vi "De_Band_HXRG.vi"(7 "Transpose":bool, 11 "IMAGE 2":i32[][](graph)=array1024x1024[1048576 elements]) -> (3 "IMAGE":dbl[][](graph))   [LabVIEW 2017]
uses:
  <vilib>/Analysis/baseanly.llb/Mean (DBL).vi
  <vilib>/Analysis/NI_AALBase.lvlib
panel:
  out "Waveform Graph 3":dbl[][](graph)
  out "Step #":i32
  out "IMAGE 3":i32[][](graph)
  out "Top Ref pixs":dbl[](array[numeric])
  out "Bottom Ref pixs":dbl[](array[numeric])
  out "Q3 avg":dbl=-0.8184616088867186
  out "Q3 RMS":dbl=19.25740971624928
  out "Q4 avg":dbl=1.3942337036132815
  out "Q4 RMS":dbl=26.97344260258525
  out "Q1 RMS":dbl=21.389760464347606
  out "Q1 avg":dbl=2.3578338623046875
  out "Q2  RMS":dbl=28.329968380841386
  out "Q2 avg":dbl=0.05986480712890625
  out "mean before":dbl=0.1424398422241211
  out "RMS before":dbl=23.67379491089448
  out "mean a fter":dbl=0.7448520660400391
  out "RMS  after":dbl=24.28217603569673
  in  "Array side Q3":u16(ring)=2 items=["Left", "Bottom", "Right", "Top"]
  in  "Array side Q4":u16(ring)=2 items=["Left", "Bottom", "Right", "Top"]
  in  "Array side Q1":u16(ring) items=["Left", "Bottom", "Right", "Top"]
  in  "Array side Q2":u16(ring) items=["Left", "Bottom", "Right", "Top"]
  out "Orig Array":i32[][](array[numeric])
  in  "Num Ref Pix":i32=5
  out "Sub Array":i32[][](array[numeric])
  # "right"
  # "left"
  # "left"
  # "right"
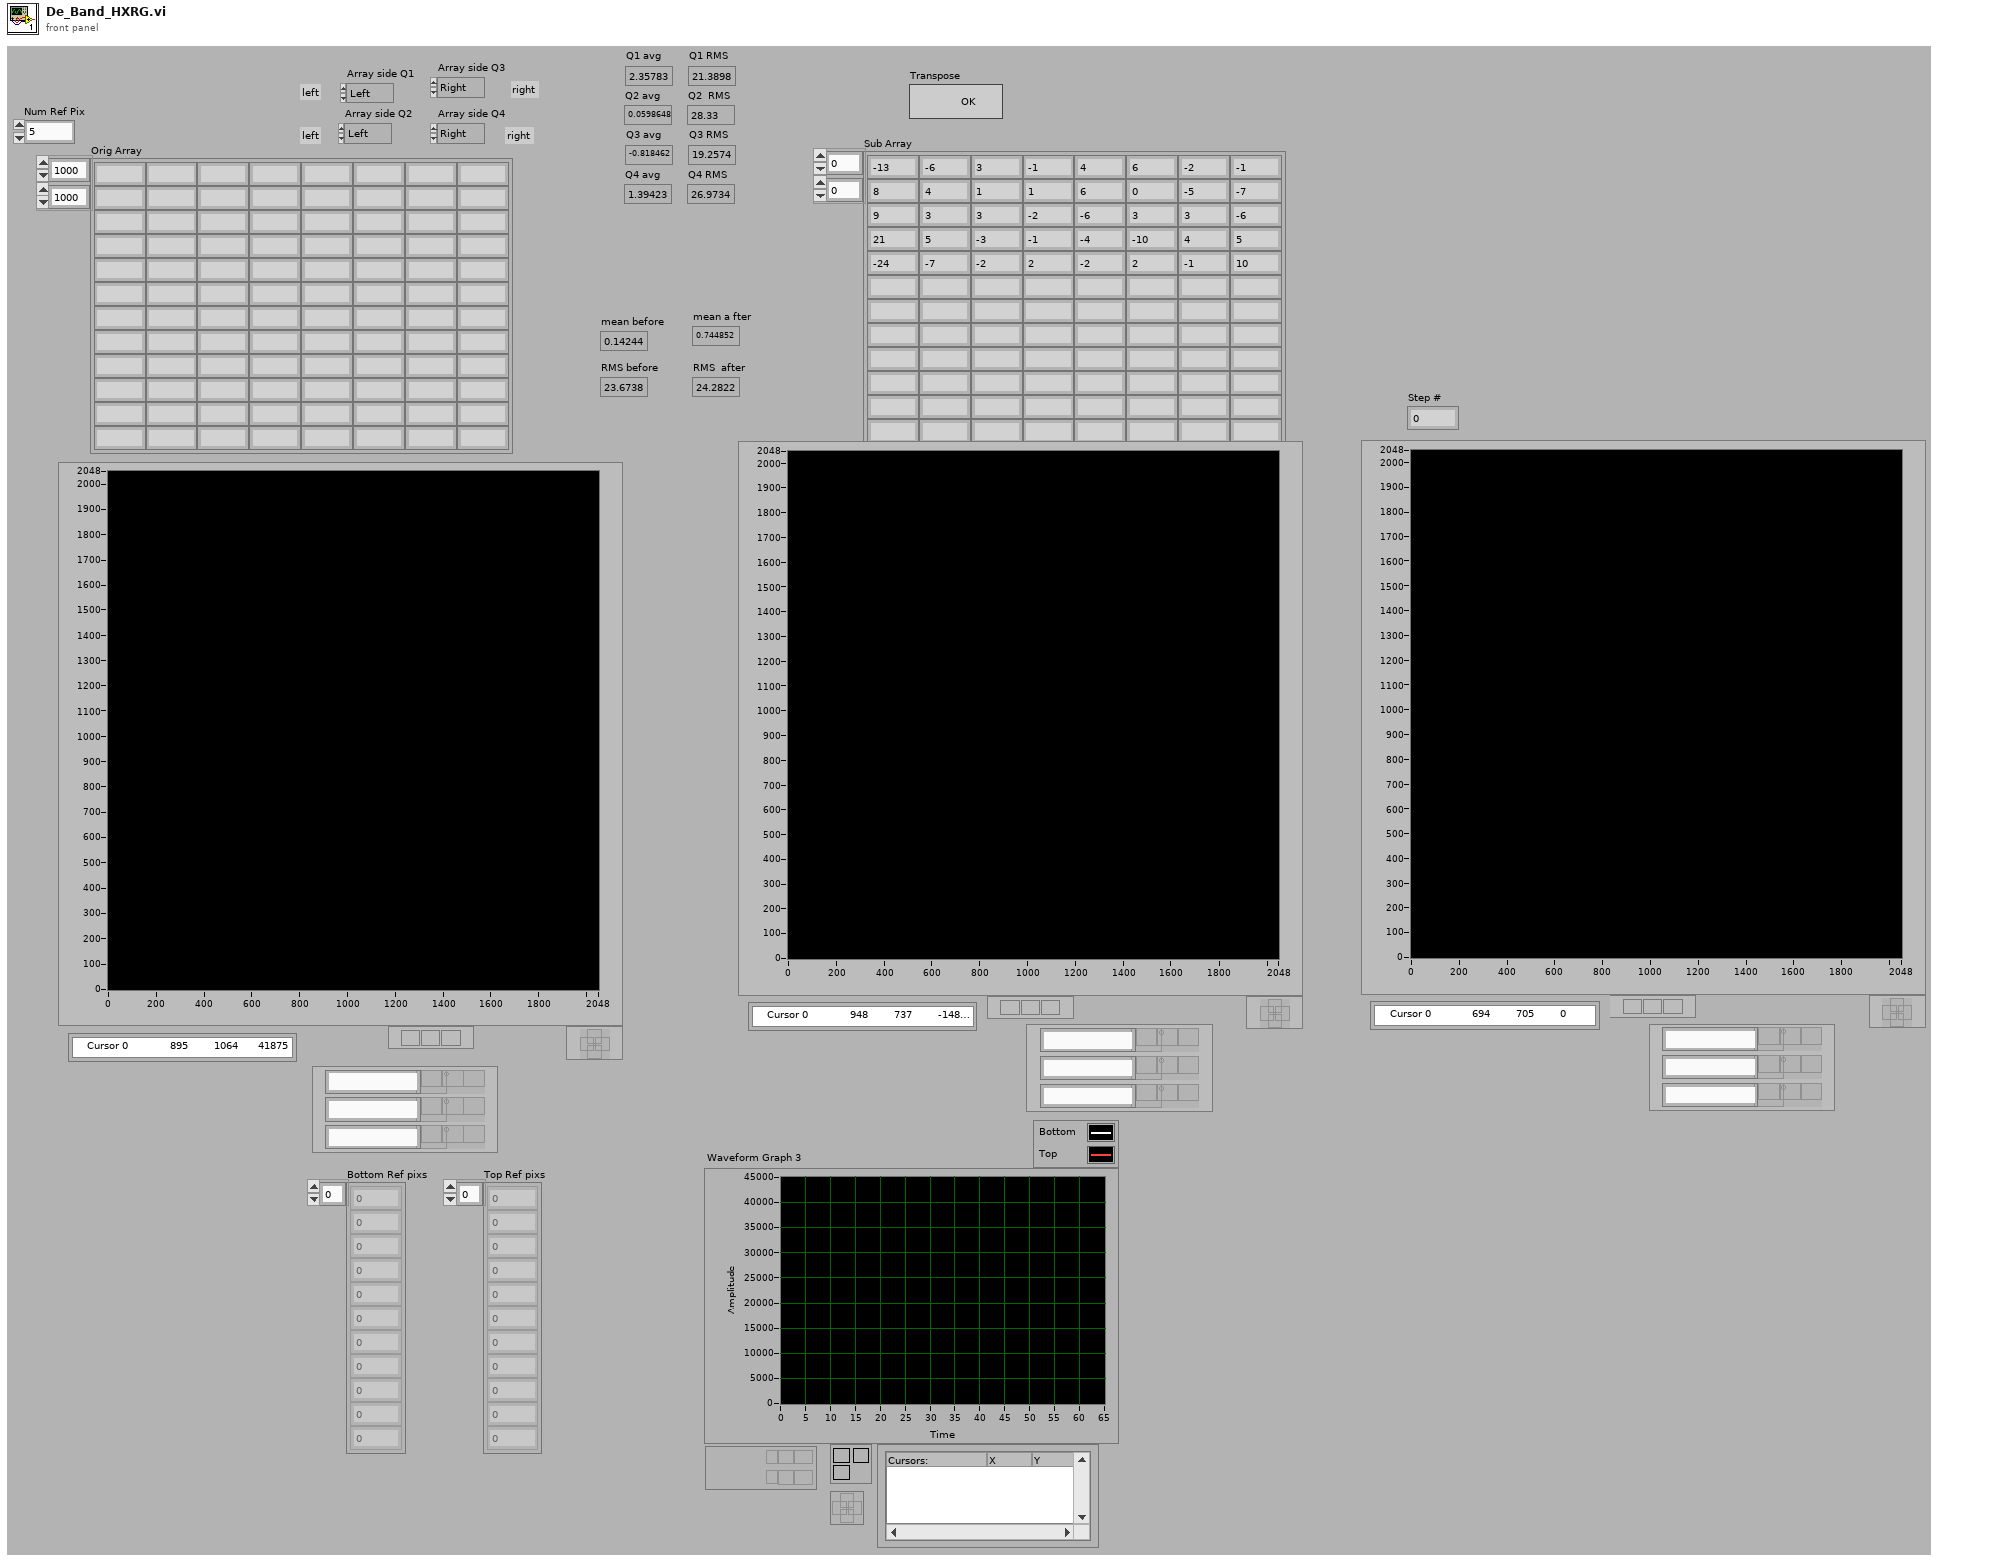
[diagram p1: front panel]
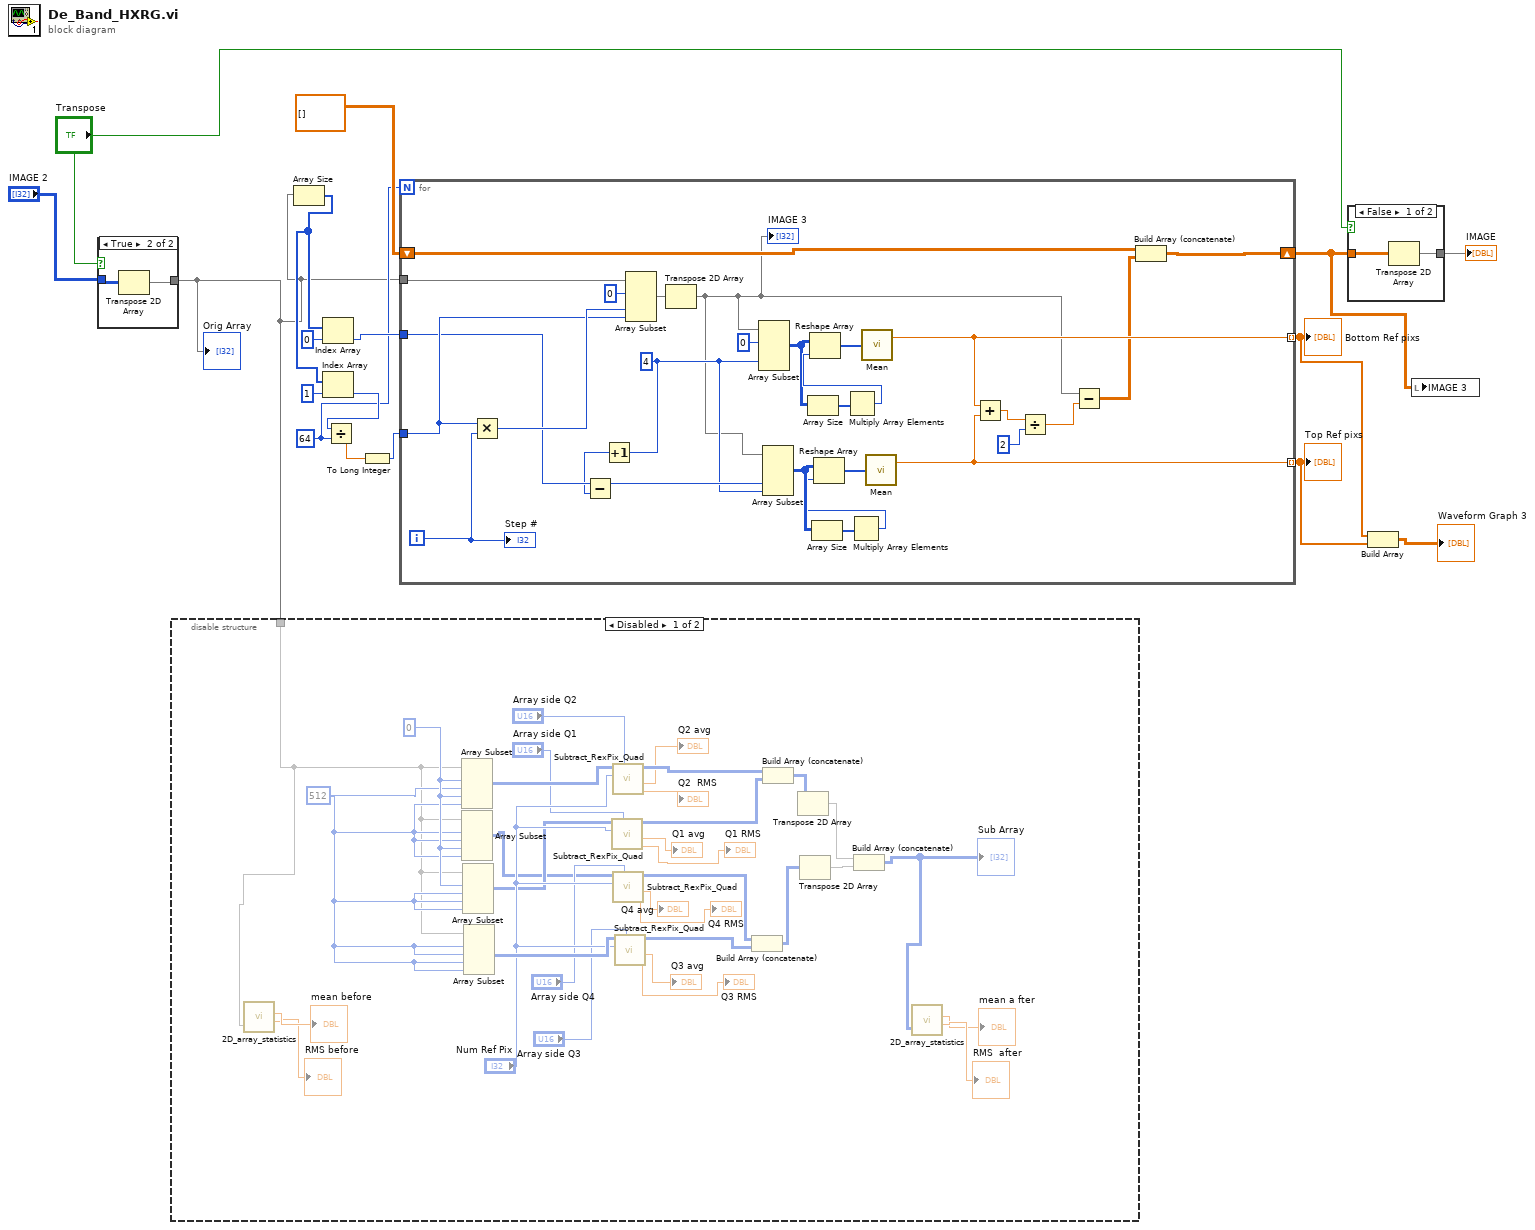
[diagram p0: block diagram]
diagram:
  w9 = 64 ("y")
  n1 = case shown="True" "Transpose" {
    tunnel: [w18 w19] -> w4
    tunnel: "IMAGE 2" -> [w18 w20]
    frame False {
    }
    frame True {
      n2 = Transpose 2D Array(2D array=w20) -> (transposed array=w19:i32[][])
    }
  }
  "Orig Array" <- w4
  n3 = disable-structure shown="Disabled" {
    disable-tunnel: w4 -> [w21 _]
    frame Disabled {
      w25 = 0
      w22 = 512
      n4 = call <userlib>:"2D_array_statistics.vi"("Array"=w21) -> ("mean 2"=→"mean before":dbl, "RMS 2"=→"RMS before":dbl)  [unwired: 2 in, 2 out]
      n5 = Array Subset(array=w21, index (row)=w25, length (row)=w22, index (col)=w25, length (col)=w22) -> (w49:i32[][])
      n6 = Array Subset(array=w21, index (row)=w22, length (row)=w22, index (col)=w25, length (col)=w22) -> (w23:i32[][])
      n7 = Array Subset(array=w21, index (row)=w25, length (row)=w22, index (col)=w22, length (col)=w22) -> (w24:i32[][])
      n8 = Array Subset(array=w21, index (row)=w22, length (row)=w22, index (col)=w22, length (col)=w22) -> (w47:i32[][])
      n9 = call <userlib>:"Subtract_RexPix_Quad.vi"("Array side"="Array side Q1", "Num Ref Pix"="Num Ref Pix", "Quad array"=w24) -> ("RMS 2"=→"Q1 RMS":dbl, "mean 2"=→"Q1 avg":dbl, "Quad array subtracted ref pixs"=w45:i32[][])  [unwired: 5 in, 1 out]
      n10 = call <userlib>:"Subtract_RexPix_Quad.vi"("Array side"="Array side Q2", "Num Ref Pix"="Num Ref Pix", "Quad array"=w49) -> ("RMS 2"=→"Q2  RMS":dbl, "mean 2"=→"Q2 avg":dbl, "Quad array subtracted ref pixs"=w48:i32[][])  [unwired: 5 in, 1 out]
      n11 = call <userlib>:"Subtract_RexPix_Quad.vi"("Array side"="Array side Q4", "Num Ref Pix"="Num Ref Pix", "Quad array"=w23) -> ("RMS 2"=→"Q4 RMS":dbl, "mean 2"=→"Q4 avg":dbl, "Quad array subtracted ref pixs"=w44:i32[][])  [unwired: 5 in, 1 out]
      n12 = call <userlib>:"Subtract_RexPix_Quad.vi"("Array side"="Array side Q3", "Num Ref Pix"="Num Ref Pix", "Quad array"=w47) -> ("RMS 2"=→"Q3 RMS":dbl, "mean 2"=→"Q3 avg":dbl, "Quad array subtracted ref pixs"=w43:i32[][])  [unwired: 5 in, 1 out]
      n13 = Build Array (concatenate)(w44, w43) -> (w50:i32[][])
      n14 = Build Array (concatenate)(w48, w45) -> (w51:i32[][])
      n15 = Transpose 2D Array(2D array=w51) -> (transposed array=w52:i32[][])
      n16 = Transpose 2D Array(2D array=w50) -> (transposed array=w53:i32[][])
      n17 = Build Array (concatenate)(w52, w53) -> (w34:i32[][])
      "Sub Array" <- w34
      n18 = call <userlib>:"2D_array_statistics.vi"("Array"=w34) -> ("mean 2"=→"mean a fter":dbl, "RMS 2"=→"RMS  after":dbl)  [unwired: 2 in, 2 out]
    }
    frame Enabled {
    }
  }
  n19 = Array Size(array=w4) -> (size(s)=w15:i32[])
  n20 = Index Array(array=w15, index=0) -> (element=w11:i32)
  n21 = Index Array(array=w15, index=1) -> (element=w14:i32)
  n22 = Divide(x=w14, y=w9) -> (x/y=w13:dbl)
  n23 = To Long Integer(number=w13) -> (32bit integer=w12:i32)
  n24 = for {
    N: w9 -> [_]
    tunnel: w4 -> [w81]
    tunnel: w12 -> [w78]
    tunnel: [w64] -> w2 mode=indexing
    tunnel: w11 -> [w68]
    tunnel: [w63] -> w3 mode=indexing
    shift-right: [w57] -> w6
    shift-left: dbl[][] [] -> [w58]
    i -> [w80]
    w66 = 4 ("length")
    n25 = Multiply(x=w78, y=w80) -> (x*y=w79:i32)
    n26 = Increment(x=w66) -> (x+1=w65:i32)
    n27 = Subtract(x=w68, y=w65) -> (x-y=w67:i32)
    n28 = Array Subset(array=w81, index (row)=0 ("index"), index (col)=w79, length (col)=w78) -> (w55:i32[][])  [unwired: 1 in]
    n29 = Transpose 2D Array(2D array=w55) -> (transposed array=w54:i32[][])
    "IMAGE 3" <- w54
    n30 = Array Subset(array=w54, index (row)=0 ("index"), length (row)=w66) -> (w73:i32[][])  [unwired: 2 in]
    n31 = Array Subset(array=w54, index (col)=w67, length (col)=w66) -> (w72:i32[][])  [unwired: 2 in]
    n32 = Array Size(array=w73) -> (size(s)=w75:i32[])
    n33 = Array Size(array=w72) -> (size(s)=w70:i32[])
    n34 = Multiply Array Elements(1:w75) -> (0:w74:i32)
    n35 = Reshape Array(w73, w74) -> (w76:i32[])
    n36 = Multiply Array Elements(1:w70) -> (0:w71:i32)
    n37 = Reshape Array(w72, w71) -> (w69:i32[])
    n38 = call-poly <vilib>:"Mean.vi"("X"=w76) -> ("mean"=w64:dbl)  [unwired: 1 out]
    n39 = call-poly <vilib>:"Mean.vi"("X"=w69) -> ("mean"=w63:dbl)  [unwired: 1 out]
    n40 = Add(x=w64, y=w63) -> (x+y=w62:dbl)
    n41 = Divide(x=w62, y=2 ("length")) -> (x/y=w60:dbl)
    n42 = Subtract(x=w54, y=w60) -> (x-y=w59:dbl[][])
    n43 = Build Array (concatenate)(w58, w59) -> (w57:dbl[][])
    "Step #" <- w80
  }
  "Bottom Ref pixs" <- w2
  "Top Ref pixs" <- w3
  n44 = case shown="False" "Transpose" {
    tunnel: w6 -> [w83 w84]
    tunnel: [w82 w84] -> w8
    frame False {
      n45 = Transpose 2D Array(2D array=w83) -> (transposed array=w82:dbl[][])
    }
    frame True {
    }
  }
  "IMAGE" <- w8
  n46 = Build Array(w2, w3) -> (→"Waveform Graph 3":dbl[][])
  n47 = local write "IMAGE 3"(w6) -> ()
